vi "Dresden R2R Sputter 03.02.2018 IY24.vi"() -> ()   [LabVIEW 2009] (continued)
                                n24994 = case shown="False" w30335 {
                                frame #0 {
                                n24995 = Wait (ms)(milliseconds to wait=u32 1000) -> ()  [unwired: 1 out]
                                n24996 = local write "SDC1 4"(TRUE ("SDC1 4")) -> ()
                                }
                                frame #1 {
                                }
                                }
                                }
                                }
                                }
                                frame #4 {
                                # "Baratron set zero"
                                n24997 = stacked-sequence {
                                frame #0 {
                                n24998 = local write "Pc_bv2_auto_baratron_set_zero"(TRUE ("Pc_bv2_auto_baratron_set_zero")) -> ()
                                }
                                frame #1 {
                                n24999 = while {
                                i -> [w30342]
                                stop <- w30339 stop-if-true
                                n25000 = Greater?(x=w30342, y=50 ("Baratron set zero time")) -> (0:w30341:bool)
                                n25001 = case shown="True" w30341 {
                                frame #0 {
                                }
                                frame #1 {
                                n25002 = local write "Semi"(TRUE ("Semi")) -> ()
                                n25003 = local write "Error Message"("" ("Error Message")) -> ()
                                }
                                }
                                n25004 = local read "Pressure 2"() -> (w30347:i32)
                                n25005 = Less?(x=w30347, y=0.1 ("Pressure Check for baratron set zero")) -> (x < y?=w30345:bool)
                                n25006 = case shown="False" w30345 {
                                tunnel: [FALSE TRUE] -> w30344
                                frame #0 {
                                n25007 = Wait Until Next ms Multiple(millisecond multiple=u32 200) -> ()  [unwired: 1 out]
                                }
                                frame #1 {
                                }
                                }
                                n25008 = local read "Semi"() -> (w30343:bool)
                                n25009 = Or(x=w30344, y=w30343) -> (x .or. y?=w30339:bool)
                                }
                                }
                                frame #2 {
                                n25010 = local read "Semi"() -> (w30353:bool)
                                n25011 = case shown="False" w30353 {
                                frame #0 {
                                n25012 = local write "SDC1 2b"(TRUE ("SDC1 2b")) -> ()
                                n25013 = Wait (ms)(milliseconds to wait=u32 1000) -> ()  [unwired: 1 out]
                                }
                                frame #1 {
                                }
                                }
                                }
                                }
                                }
                                frame #5 {
                                # "CC CLOSE"
                                n25014 = stacked-sequence {
                                frame #0 {
                                n25015 = local read "Semi"() -> (w30356:bool)
                                n25016 = case shown="False" w30356 {
                                frame #0 {
                                n25017 = while {
                                i -> [w30362]
                                stop <- w30357 stop-if-true
                                n25018 = Greater?(x=w30362, y=50) -> (0:w30361:bool)
                                n25019 = case shown="True" w30361 {
                                frame #0 {
                                }
                                frame #1 {
                                n25020 = local write "Semi"(TRUE ("Semi")) -> ()
                                n25021 = local write "Error Message"("Coating Process  \nwas cancelled.\nPlease check \nBG-BV connection." ("Error Message")) -> ()
                                }
                                }
                                n25022 = local read "Ch2_Cc_on_off_di"() -> (w30360:bool)
                                n25023 = case shown="True" w30360 {
                                tunnel: [TRUE FALSE] -> w30359
                                frame #0 {
                                }
                                frame #1 {
                                n25024 = local write "Ch2_Cc_on_off_do"(FALSE ("Ch1_WFC_do")) -> ()
                                n25025 = Wait Until Next ms Multiple(millisecond multiple=u32 200) -> ()  [unwired: 1 out]
                                }
                                }
                                n25026 = local read "Semi"() -> (w30358:bool)
                                n25027 = Or(x=w30359, y=w30358) -> (x .or. y?=w30357:bool)
                                }
                                }
                                frame #1 {
                                }
                                }
                                }
                                frame #1 {
                                n25028 = local read "Semi"() -> (w30370:bool)
                                n25029 = case shown="False" w30370 {
                                frame #0 {
                                n25030 = local write "SDC1 3"(TRUE ("SDC1 3")) -> ()
                                n25031 = Wait (ms)(milliseconds to wait=u32 1000) -> ()  [unwired: 1 out]
                                }
                                frame #1 {
                                }
                                }
                                }
                                }
                                }
                                frame #6 {
                                # "PC-BV CLOSE"
                                n25032 = stacked-sequence {
                                frame #0 {
                                n25033 = local read "Semi"() -> (w30373:bool)
                                n25034 = case shown="False" w30373 {
                                frame #0 {
                                n25035 = stacked-sequence {
                                frame #0 {
                                n25036 = local read "Semi"() -> (w30374:bool)
                                n25037 = case shown="False" w30374 {
                                frame #0 {
                                n25038 = local write "Pc_bv2_auto_close"(TRUE ("Tp1_auto_start")) -> ()
                                }
                                frame #1 {
                                }
                                }
                                }
                                frame #1 {
                                n25039 = local read "Semi"() -> (w30376:bool)
                                n25040 = case shown="False" w30376 {
                                frame #0 {
                                n25041 = Wait (ms)(milliseconds to wait=u32 1000) -> ()  [unwired: 1 out]
                                }
                                frame #1 {
                                }
                                }
                                }
                                frame #2 {
                                n25042 = local read "Semi"() -> (w30378:bool)
                                n25043 = case shown="False" w30378 {
                                frame #0 {
                                n25044 = while {
                                i -> [w30384]
                                stop <- w30380 stop-if-true
                                n25045 = local read "Pc_bv_closed_ch2"() -> (w30382:bool)
                                n25046 = Greater?(x=w30384, y=120) -> (0:w30383:bool)
                                n25047 = local read "Semi"() -> (w30381:bool)
                                n25048 = Compound Arithmetic op=OR(w30381, w30382, w30383) -> (w30380:bool)
                                n25049 = Wait (ms)(milliseconds to wait=u32 500) -> ()  [unwired: 1 out]
                                }
                                }
                                frame #1 {
                                }
                                }
                                }
                                frame #3 {
                                n25050 = local read "Semi"() -> (w30386:bool)
                                n25051 = case shown="False" w30386 {
                                frame #0 {
                                n25052 = local read "Pc_bv_closed_ch2"() -> (w30387:bool)
                                n25053 = case shown="False" w30387 {
                                frame #0 {
                                n25054 = local write "Pc_bv2_auto_close"(TRUE ("Pc_bv1_auto_open")) -> ()
                                }
                                frame #1 {
                                }
                                }
                                }
                                frame #1 {
                                }
                                }
                                }
                                frame #4 {
                                n25055 = local read "Semi"() -> (w30389:bool)
                                n25056 = case shown="False" w30389 {
                                frame #0 {
                                n25057 = local read "Pc_bv_closed_ch2"() -> (w30390:bool)
                                n25058 = case shown="False" w30390 {
                                frame #0 {
                                n25059 = Wait (ms)(milliseconds to wait=u32 1000) -> ()  [unwired: 1 out]
                                }
                                frame #1 {
                                }
                                }
                                }
                                frame #1 {
                                }
                                }
                                }
                                frame #5 {
                                n25060 = local read "Semi"() -> (w30392:bool)
                                n25061 = case shown="False" w30392 {
                                frame #0 {
                                n25062 = while {
                                i -> [w30398]
                                stop <- w30394 stop-if-true
                                n25063 = local read "Pc_bv_closed_ch2"() -> (w30396:bool)
                                n25064 = Greater?(x=w30398, y=120) -> (0:w30397:bool)
                                n25065 = local read "Semi"() -> (w30395:bool)
                                n25066 = Compound Arithmetic op=OR(w30395, w30396, w30397) -> (w30394:bool)
                                n25067 = Wait (ms)(milliseconds to wait=u32 500) -> ()  [unwired: 1 out]
                                }
                                }
                                frame #1 {
                                }
                                }
                                }
                                frame #6 {
                                n25068 = local read "Semi"() -> (w30400:bool)
                                n25069 = case shown="False" w30400 {
                                frame #0 {
                                n25070 = local read "Pc_bv_closed_ch2"() -> (w30401:bool)
                                n25071 = case shown="False" w30401 {
                                frame #0 {
                                n25072 = local write "Error Message"("Start up process  cancelled\nbecause  PC-BV not closed.\nPlease check PC-BV1 connections." ("Error Message")) -> ()
                                n25073 = Wait (ms)(milliseconds to wait=u32 1000) -> ()  [unwired: 1 out]
                                }
                                frame #1 {
                                }
                                }
                                }
                                frame #1 {
                                }
                                }
                                }
                                }
                                }
                                frame #1 {
                                }
                                }
                                }
                                frame #1 {
                                n25074 = local read "Semi"() -> (w30404:bool)
                                n25075 = case shown="False" w30404 {
                                frame #0 {
                                n25076 = local write "SDC1 5"(TRUE ("SDC1 5")) -> ()
                                n25077 = Wait (ms)(milliseconds to wait=u32 1000) -> ()  [unwired: 1 out]
                                }
                                frame #1 {
                                }
                                }
                                }
                                }
                                }
                                frame #7 {
                                # "SOV-AR OPEN"
                                n25078 = stacked-sequence {
                                frame #0 {
                                n25079 = local read "Semi"() -> (w30407:bool)
                                n25080 = case shown="False" w30407 {
                                frame #0 {
                                n25081 = while {
                                i -> [w30413]
                                stop <- w30408 stop-if-true
                                n25082 = Greater?(x=w30413, y=50) -> (0:w30412:bool)
                                n25083 = case shown="True" w30412 {
                                frame #0 {
                                }
                                frame #1 {
                                n25084 = local write "Semi"(TRUE ("Semi")) -> ()
                                n25085 = local write "Error Message"("Coating Process  \nwas cancelled.\nPlease check \nSOV-Ar connection." ("Error Message")) -> ()
                                }
                                }
                                n25086 = local read "Ch2_Sov_Ar_di"() -> (w30411:bool)
                                n25087 = case shown="False" w30411 {
                                tunnel: [FALSE TRUE] -> w30410
                                frame #0 {
                                n25088 = local write "Ch2_Sov_Ar_do"(TRUE ("Ch1_WFC_do")) -> ()
                                n25089 = Wait Until Next ms Multiple(millisecond multiple=u32 200) -> ()  [unwired: 1 out]
                                }
                                frame #1 {
                                }
                                }
                                n25090 = local read "Semi"() -> (w30409:bool)
                                n25091 = Or(x=w30410, y=w30409) -> (x .or. y?=w30408:bool)
                                }
                                }
                                frame #1 {
                                }
                                }
                                }
                                frame #1 {
                                n25092 = local read "Semi"() -> (w30421:bool)
                                n25093 = case shown="False" w30421 {
                                frame #0 {
                                n25094 = while {
                                i -> [w30426]
                                stop <- w30424 stop-if-true
                                n25095 = Greater?(x=w30426, y=5) -> (0:w30422:bool)
                                n25096 = Wait Until Next ms Multiple(millisecond multiple=u32 1000) -> ()  [unwired: 1 out]
                                n25097 = local read "Semi"() -> (w30425:bool)
                                n25098 = Or(x=w30422, y=w30425) -> (x .or. y?=w30424:bool)
                                }
                                }
                                frame #1 {
                                }
                                }
                                }
                                frame #2 {
                                n25099 = local read "Semi"() -> (w30428:bool)
                                n25100 = case shown="False" w30428 {
                                frame #0 {
                                n25101 = local write "SDC1 6"(TRUE ("SDC1 6")) -> ()
                                n25102 = Wait (ms)(milliseconds to wait=u32 1000) -> ()  [unwired: 1 out]
                                }
                                frame #1 {
                                }
                                }
                                }
                                }
                                }
                                frame #8 {
                                # "CHECK CHAMBER PRESSURE"
                                n25103 = stacked-sequence {
                                frame #0 {
                                n25104 = local read "Semi"() -> (w30431:bool)
                                n25105 = case shown="False" w30431 {
                                frame #0 {
                                n25106 = while {
                                i -> [w30439]
                                stop <- w30433 stop-if-true
                                n25107 = Greater?(x=w30439, y=300) -> (0:w30438:bool)
                                n25108 = case shown="True" w30438 {
                                frame #0 {
                                }
                                frame #1 {
                                n25109 = local write "Semi"(TRUE ("Semi")) -> ()
                                n25110 = local write "Error Message"("Coating Process cancelled.\nPlease check chamber \nconnections." ("Error Message")) -> ()
                                }
                                }
                                n25111 = local read "Ch_pg_press_ch2_gui 2"() -> (w30432:dbl)
                                n25112 = Greater Or Equal?(x=w30432, y=0.9 ("CHAMBER PRESSURE 4")) -> (x >= y?=w30436:bool)
                                n25113 = case shown="True" w30436 {
                                tunnel: [TRUE FALSE] -> w30435
                                frame #0 {
                                }
                                frame #1 {
                                n25114 = Wait Until Next ms Multiple(millisecond multiple=u32 200) -> ()  [unwired: 1 out]
                                }
                                }
                                n25115 = local read "Semi"() -> (w30434:bool)
                                n25116 = Or(x=w30435, y=w30434) -> (x .or. y?=w30433:bool)
                                }
                                }
                                frame #1 {
                                }
                                }
                                }
                                frame #1 {
                                n25117 = local read "Semi"() -> (w30446:bool)
                                n25118 = case shown="False" w30446 {
                                frame #0 {
                                n25119 = Wait (ms)(milliseconds to wait=u32 1000) -> ()  [unwired: 1 out]
                                n25120 = local write "SDC1 8"(TRUE ("SDC1 8")) -> ()
                                }
                                frame #1 {
                                }
                                }
                                }
                                }
                                }
                                frame #9 {
                                # "PC-BV OPEN"
                                n25121 = stacked-sequence {
                                frame #0 {
                                n25122 = local read "Semi"() -> (w30449:bool)
                                n25123 = case shown="False" w30449 {
                                frame #0 {
                                n25124 = stacked-sequence {
                                frame #0 {
                                n25125 = local read "Semi"() -> (w30450:bool)
                                n25126 = case shown="False" w30450 {
                                frame #0 {
                                n25127 = local write "Pc_bv2_auto_open"(TRUE ("Tp1_auto_start")) -> ()
                                }
                                frame #1 {
                                }
                                }
                                }
                                frame #1 {
                                n25128 = local read "Semi"() -> (w30452:bool)
                                n25129 = case shown="False" w30452 {
                                frame #0 {
                                n25130 = Wait (ms)(milliseconds to wait=u32 1000) -> ()  [unwired: 1 out]
                                }
                                frame #1 {
                                }
                                }
                                }
                                frame #2 {
                                n25131 = local read "Semi"() -> (w30454:bool)
                                n25132 = case shown="False" w30454 {
                                frame #0 {
                                n25133 = while {
                                i -> [w30460]
                                stop <- w30456 stop-if-true
                                n25134 = local read "Pc_bv_opened_ch2"() -> (w30458:bool)
                                n25135 = Greater?(x=w30460, y=120) -> (0:w30459:bool)
                                n25136 = local read "Semi"() -> (w30457:bool)
                                n25137 = Compound Arithmetic op=OR(w30457, w30458, w30459) -> (w30456:bool)
                                n25138 = Wait (ms)(milliseconds to wait=u32 500) -> ()  [unwired: 1 out]
                                }
                                }
                                frame #1 {
                                }
                                }
                                }
                                frame #3 {
                                n25139 = local read "Semi"() -> (w30462:bool)
                                n25140 = case shown="False" w30462 {
                                frame #0 {
                                n25141 = local read "Pc_bv_opened_ch2"() -> (w30463:bool)
                                n25142 = case shown="False" w30463 {
                                frame #0 {
                                n25143 = local write "Pc_bv2_auto_open"(TRUE ("Pc_bv1_auto_open")) -> ()
                                }
                                frame #1 {
                                }
                                }
                                }
                                frame #1 {
                                }
                                }
                                }
                                frame #4 {
                                n25144 = local read "Semi"() -> (w30465:bool)
                                n25145 = case shown="False" w30465 {
                                frame #0 {
                                n25146 = local read "Pc_bv_opened_ch2"() -> (w30466:bool)
                                n25147 = case shown="False" w30466 {
                                frame #0 {
                                n25148 = Wait (ms)(milliseconds to wait=u32 1000) -> ()  [unwired: 1 out]
                                }
                                frame #1 {
                                }
                                }
                                }
                                frame #1 {
                                }
                                }
                                }
                                frame #5 {
                                n25149 = local read "Semi"() -> (w30468:bool)
                                n25150 = case shown="False" w30468 {
                                frame #0 {
                                n25151 = while {
                                i -> [w30474]
                                stop <- w30470 stop-if-true
                                n25152 = local read "Pc_bv_opened_ch2"() -> (w30472:bool)
                                n25153 = Greater?(x=w30474, y=120) -> (0:w30473:bool)
                                n25154 = local read "Semi"() -> (w30471:bool)
                                n25155 = Compound Arithmetic op=OR(w30471, w30472, w30473) -> (w30470:bool)
                                n25156 = Wait (ms)(milliseconds to wait=u32 500) -> ()  [unwired: 1 out]
                                }
                                }
                                frame #1 {
                                }
                                }
                                }
                                frame #6 {
                                n25157 = local read "Semi"() -> (w30476:bool)
                                n25158 = case shown="False" w30476 {
                                frame #0 {
                                n25159 = local read "Pc_bv_opened_ch2"() -> (w30477:bool)
                                n25160 = case shown="False" w30477 {
                                frame #0 {
                                n25161 = local write "Error Message"("Start up process  cancelled\nbecause  PC-BV not opened.\nPlease check PC-BV1 connections." ("Error Message")) -> ()
                                n25162 = Wait (ms)(milliseconds to wait=u32 1000) -> ()  [unwired: 1 out]
                                }
                                frame #1 {
                                }
                                }
                                }
                                frame #1 {
                                }
                                }
                                }
                                }
                                }
                                frame #1 {
                                }
                                }
                                }
                                frame #1 {
                                n25163 = local read "Semi"() -> (w30480:bool)
                                n25164 = case shown="False" w30480 {
                                frame #0 {
                                n25165 = Wait (ms)(milliseconds to wait=u32 1000) -> ()  [unwired: 1 out]
                                n25166 = local write "SDC1 7"(TRUE ("SDC1 7")) -> ()
                                }
                                frame #1 {
                                }
                                }
                                }
                                }
                                }
                                frame #10 {
                                # "CC OPEN"
                                n25167 = stacked-sequence {
                                frame #0 {
                                n25168 = local read "Semi"() -> (w30483:bool)
                                n25169 = case shown="False" w30483 {
                                frame #0 {
                                n25170 = while {
                                i -> [w30489]
                                stop <- w30484 stop-if-true
                                n25171 = Greater?(x=w30489, y=50) -> (0:w30488:bool)
                                n25172 = case shown="True" w30488 {
                                frame #0 {
                                }
                                frame #1 {
                                n25173 = local write "Semi"(TRUE ("Semi")) -> ()
                                n25174 = local write "Error Message"("Coating Process  \nwas cancelled.\nPlease check \nBG-BV connection." ("Error Message")) -> ()
                                }
                                }
                                n25175 = local read "Ch2_Cc_on_off_di"() -> (w30487:bool)
                                n25176 = case shown="True" w30487 {
                                tunnel: [FALSE TRUE] -> w30486
                                frame #0 {
                                n25177 = local write "Ch2_Cc_on_off_do"(TRUE ("Ch1_WFC_do")) -> ()
                                n25178 = Wait Until Next ms Multiple(millisecond multiple=u32 200) -> ()  [unwired: 1 out]
                                }
                                frame #1 {
                                }
                                }
                                n25179 = local read "Semi"() -> (w30485:bool)
                                n25180 = Or(x=w30486, y=w30485) -> (x .or. y?=w30484:bool)
                                }
                                }
                                frame #1 {
                                }
                                }
                                }
                                frame #1 {
                                n25181 = local read "Semi"() -> (w30497:bool)
                                n25182 = case shown="False" w30497 {
                                frame #0 {
                                n25183 = while {
                                i -> [w30502]
                                stop <- w30500 stop-if-true
                                n25184 = Greater?(x=w30502, y=30) -> (0:w30498:bool)
                                n25185 = Wait Until Next ms Multiple(millisecond multiple=u32 1000) -> ()  [unwired: 1 out]
                                n25186 = local read "Semi"() -> (w30501:bool)
                                n25187 = Or(x=w30498, y=w30501) -> (x .or. y?=w30500:bool)
                                }
                                }
                                frame #1 {
                                }
                                }
                                }
                                frame #2 {
                                n25188 = local read "Semi"() -> (w30504:bool)
                                n25189 = case shown="False" w30504 {
                                frame #0 {
                                n25190 = Wait (ms)(milliseconds to wait=u32 1000) -> ()  [unwired: 1 out]
                                n25191 = local write "SDC1 7b"(TRUE ("SDC1 3")) -> ()
                                }
                                frame #1 {
                                }
                                }
                                }
                                }
                                }
                                frame #11 {
                                # "CHECK CHAMBER PRESSURE"
                                n25192 = stacked-sequence {
                                frame #0 {
                                n25193 = local read "Semi"() -> (w30507:bool)
                                n25194 = case shown="False" w30507 {
                                frame #0 {
                                n25195 = while {
                                i -> [w30515]
                                stop <- w30509 stop-if-true
                                n25196 = Greater?(x=w30515, y=300) -> (0:w30514:bool)
                                n25197 = case shown="True" w30514 {
                                frame #0 {
                                }
                                frame #1 {
                                n25198 = local write "Semi"(TRUE ("Semi")) -> ()
                                n25199 = local write "Error Message"("Coating Process cancelled.\nPlease check chamber \nconnections." ("Error Message")) -> ()
                                }
                                }
                                n25200 = local read "Ch_CC_press_ch2 2"() -> (w30508:dbl)
                                n25201 = Greater Or Equal?(x=w30508, y=5e-05 ("CHAMBER PRESSURE 5")) -> (x >= y?=w30512:bool)
                                n25202 = case shown="True" w30512 {
                                tunnel: [TRUE FALSE] -> w30511
                                frame #0 {
                                }
                                frame #1 {
                                n25203 = Wait Until Next ms Multiple(millisecond multiple=u32 200) -> ()  [unwired: 1 out]
                                }
                                }
                                n25204 = local read "Semi"() -> (w30510:bool)
                                n25205 = Or(x=w30511, y=w30510) -> (x .or. y?=w30509:bool)
                                }
                                }
                                frame #1 {
                                }
                                }
                                }
                                frame #1 {
                                n25206 = local read "Semi"() -> (w30522:bool)
                                n25207 = case shown="False" w30522 {
                                frame #0 {
                                n25208 = Wait (ms)(milliseconds to wait=u32 1000) -> ()  [unwired: 1 out]
                                n25209 = local write "SDC1 10"(TRUE ("SDC1 10")) -> ()
                                }
                                frame #1 {
                                }
                                }
                                }
                                }
                                }
                                frame #12 {
                                # "CC CLOSE"
                                n25210 = stacked-sequence {
                                frame #0 {
                                n25211 = local read "Semi"() -> (w30525:bool)
                                n25212 = case shown="False" w30525 {
                                frame #0 {
                                n25213 = while {
                                i -> [w30531]
                                stop <- w30526 stop-if-true
                                n25214 = Greater?(x=w30531, y=50) -> (0:w30530:bool)
                                n25215 = case shown="True" w30530 {
                                frame #0 {
                                }
                                frame #1 {
                                n25216 = local write "Semi"(TRUE ("Semi")) -> ()
                                n25217 = local write "Error Message"("Coating Process  \nwas cancelled.\nPlease check \nBG-BV connection." ("Error Message")) -> ()
                                }
                                }
                                n25218 = local read "Ch2_Cc_on_off_di"() -> (w30529:bool)
                                n25219 = case shown="True" w30529 {
                                tunnel: [TRUE FALSE] -> w30528
                                frame #0 {
                                }
                                frame #1 {
                                n25220 = local write "Ch2_Cc_on_off_do"(FALSE ("Ch1_WFC_do")) -> ()
                                n25221 = Wait Until Next ms Multiple(millisecond multiple=u32 200) -> ()  [unwired: 1 out]
                                }
                                }
                                n25222 = local read "Semi"() -> (w30527:bool)
                                n25223 = Or(x=w30528, y=w30527) -> (x .or. y?=w30526:bool)
                                }
                                }
                                frame #1 {
                                }
                                }
                                }
                                frame #1 {
                                n25224 = local read "Semi"() -> (w30539:bool)
                                n25225 = case shown="False" w30539 {
                                frame #0 {
                                n25226 = local write "SDC1 10b"(TRUE ("SDC1 3")) -> ()
                                n25227 = Wait (ms)(milliseconds to wait=u32 1000) -> ()  [unwired: 1 out]
                                }
                                frame #1 {
                                }
                                }
                                }
                                }
                                }
                                frame #13 {
                                # "SET Ar FLOW"
                                n25228 = local read "R_Web_selection"() -> (w30542:enum32{"Web", "Other"})
                                n25229 = case shown="\"Other\"" w30542 {
                                frame #0 {
                                }
                                frame #1 {
                                n25230 = stacked-sequence {
                                frame #0 {
                                n25231 = local read "Semi"() -> (w30543:bool)
                                n25232 = case shown="False" w30543 {
                                frame #0 {
                                n25233 = stacked-sequence {
                                frame #0 {
                                n25234 = local read "Semi"() -> (w30544:bool)
                                n25235 = case shown="False" w30544 {
                                frame #0 {
                                n25236 = local read "R Argon Flow sccm"() -> (w30545:dbl)
                                n25237 = local write "Ar_sccm1_2"(w30545) -> ()
                                }
                                frame #1 {
                                }
                                }
                                }
                                frame #1 {
                                n25238 = local read "Semi"() -> (w30546:bool)
                                n25239 = case shown="False" w30546 {
                                frame #0 {
                                n25240 = local write "Mfc_Ar _1_2_set"(TRUE ("Mfc_Ar _1_2_set")) -> ()
                                }
                                frame #1 {
                                }
                                }
                                }
                                frame #2 {
                                n25241 = local read "Semi"() -> (w30548:bool)
                                n25242 = case shown="False" w30548 {
                                frame #0 {
                                n25243 = while {
                                i -> [w30551]
                                stop <- w30553 stop-if-true
                                n25244 = Greater?(x=w30551, y=50) -> (0:w30550:bool)
                                n25245 = local read "Semi"() -> (w30549:bool)
                                n25246 = Or(x=w30549, y=w30550) -> (x .or. y?=w30553:bool)
                                }
                                }
                                frame #1 {
                                }
                                }
                                }
                                frame #3 {
                                n25247 = local read "Semi"() -> (w30554:bool)
                                n25248 = case shown="False" w30554 {
                                frame #0 {
                                n25249 = local read "Ar_sccm_act 6"() -> (w30555:dbl)
                                n25250 = Greater?(x=w30555, y=1) -> (0:w30556:bool)
                                n25251 = case shown="False" w30556 {
                                frame #0 {
                                n25252 = local read "R Argon Flow sccm"() -> (w30558:dbl)
                                n25253 = local write "Ar_sccm1_2"(w30558) -> ()
                                }
                                frame #1 {
                                }
                                }
                                }
                                frame #1 {
                                }
                                }
                                }
                                frame #4 {
                                n25254 = local read "Semi"() -> (w30559:bool)
                                n25255 = case shown="False" w30559 {
                                frame #0 {
                                n25256 = local read "Ar_sccm_act 6"() -> (w30561:dbl)
                                n25257 = Greater?(x=w30561, y=1) -> (0:w30560:bool)
                                n25258 = case shown="False" w30560 {
                                frame #0 {
                                n25259 = while {
                                i -> [w30564]
                                stop <- w30568 stop-if-true
                                n25260 = Greater?(x=w30564, y=50) -> (0:w30563:bool)
                                n25261 = local read "Semi"() -> (w30567:bool)
                                n25262 = case shown="False" w30567 {
                                tunnel: [FALSE TRUE] -> w30566
                                frame #0 {
                                n25263 = Wait Until Next ms Multiple(millisecond multiple=u32 200) -> ()  [unwired: 1 out]
                                }
                                frame #1 {
                                }
                                }
                                n25264 = Or(x=w30566, y=w30563) -> (x .or. y?=w30568:bool)
                                }
                                }
                                frame #1 {
                                }
                                }
                                }
                                frame #1 {
                                }
                                }
                                }
                                frame #5 {
                                n25265 = local read "Semi"() -> (w30572:bool)
                                n25266 = case shown="False" w30572 {
                                frame #0 {
                                n25267 = local read "Ar_sccm_act 5"() -> (w30574:dbl)
                                n25268 = Greater?(x=w30574, y=1) -> (0:w30573:bool)
                                n25269 = case shown="False" w30573 {
                                frame #0 {
                                n25270 = local write "Semi"(TRUE ("Semi")) -> ()
                                n25271 = local write "Error Message"("Coating process cancelled.\nPlease check connections." ("Error Message")) -> ()
                                }
                                frame #1 {
                                }
                                }
                                }
                                frame #1 {
                                }
                                }
                                }
                                }
                                }
                                frame #1 {
                                }
                                }
                                }
                                frame #1 {
                                n25272 = local read "Semi"() -> (w30578:bool)
                                n25273 = case shown="False" w30578 {
                                frame #0 {
                                n25274 = local write "SDC1 11"(TRUE ("SDC1 11")) -> ()
                                n25275 = Wait (ms)(milliseconds to wait=u32 1000) -> ()  [unwired: 1 out]
                                }
                                frame #1 {
                                }
                                }
                                }
                                }
                                }
                                }
                                }
                                frame #14 {
                                # "Set  Pressure"
                                n25276 = local read "R_Web_selection"() -> (w30581:enum32{"Web", "Other"})
                                n25277 = case shown="\"Other\"" w30581 {
                                frame #0 {
                                }
                                frame #1 {
                                n25278 = stacked-sequence {
                                frame #0 {
                                n25279 = local read "Semi"() -> (w30582:bool)
                                n25280 = case shown="False" w30582 {
                                frame #0 {
                                n25281 = stacked-sequence {
                                frame #0 {
                                n25282 = local read "Semi"() -> (w30583:bool)
                                n25283 = case shown="False" w30583 {